vi "UHR-Fleezers Control (host) - 12.8.1.vi"() -> ()   [LabVIEW 2012] (continued)
      }
    }
    n3050 = Negate(x=w3835) -> (-x=w3648:dbl[])
    n3051 = Subtract(x=w3648, y="Offset (nm)") -> (x-y=w3809:dbl[])
    n3052 = case "Choose calibrated display" shown="2" "Calibration" {
      tunnel: w3579 -> [w4240 _ _]
      tunnel: w3576 -> [w4239 _ _]
      tunnel: [w4240 w4242 w4244] -> w3848
      tunnel: [w4239 w4241 w4243] -> w3847
      tunnel: w3578 -> [_ w4242 _]
      tunnel: w3577 -> [_ _ w4244]
      tunnel: w3575 -> [_ w4241 _]
      tunnel: w3574 -> [_ _ w4243]
      frame 0, Default {
      }
      frame 1 {
      }
      frame 2 {
      }
    }
    n3053 = Bundle By Name(cluster=w3579, "Y"=w3809) -> (w3573:waveform(dbl))
    "Bead Separation" <- w3573
    n3054 = feedback #24(w3809) -> (w3808:dbl[])
    n3055 = Build Array (concatenate)(w3809, w3808) -> (w3585:dbl[])
    n3056 = Split 1D Array(array=w3585, index=w3708) -> (first subarray=w3586:dbl[])  [unwired: 1 out]
    n3057 = feedback-in #24(w3586) -> ()
    n3058 = Build Array(w3579, w3578, w3577, w3576, w3575, w3574, w3573) -> (w3572:waveform(dbl)[])
    n3059 = Not(x="Trap Trig. Fl.") -> (.not. x?=w3684:bool)
    n3060 = Unbundle By Name(w3848) -> ("Y"=w3649:dbl[])
    n3061 = Unbundle By Name(w3847) -> ("Y"=w3810:dbl[])
    n3062 = call-poly <vilib>:"Mean.vi"("X"=w3586) -> ("mean"=w3805:dbl)  [unwired: 1 out]
    "Bead Mean (nm)" <- w3805
    n3063 = Multiply(x=w3847, y=-1.0) -> (x*y=w3837:waveform(dbl))
    n3064 = call-poly <vilib>:"Mean.vi"("X"=w3649) -> ("mean"=w3652:dbl)  [unwired: 1 out]
    "T1 X" <- w3652
    n3065 = call-poly <vilib>:"Mean.vi"("X"=w3810) -> ("mean"=w3651:dbl)  [unwired: 1 out]
    "T2 X" <- w3651
    n3066 = Build Array(w3848, w3837) -> (→"Force":waveform(dbl)[])
    n3067 = Subtract(x=w3586, y=w3805) -> (x-y=w3804:dbl[])
    n3068 = Square(x=w3804) -> (x^2=w3803:dbl[])
    n3069 = Negate(x=w3810) -> (-x=w3598:dbl[])
    n3070 = call-poly <vilib>:"Mean.vi"("X"=w3803) -> ("mean"=w3802:dbl)  [unwired: 1 out]
    n3071 = Negate(x=w3651) -> (-x=w3650:dbl)
    n3072 = Square Root(x=w3802) -> (sqrt(x)=w3801:dbl)
    n3073 = Add(x=w3649, y=w3598) -> (x+y=w3811:dbl[])
    n3074 = Add(x=w3652, y=w3650) -> (x+y=w3842:dbl)
    n3075 = Multiply(x=10.0, y=w3801) -> (x*y=→"RMS (Ang)":dbl)
    n3076 = Divide(x=w3811, y=2.0) -> (x/y=w3601:dbl[])
    n3077 = Subtract(x=w3652, y=w3650) -> (x-y=→"Difference":dbl)
    n3078 = Select(t=w3598, s="Only check fixed trap T2", f=w3601) -> (s? t:f=→"Vec Mean of T1 T2":dbl[])
    n3079 = Divide(x=w3842, y=2.0) -> (x/y=w3813:dbl)
    "Mean" <- w3813
    n3080 = feedback-in #25("Trap Trig. Fl.") -> ()
    n3081 = feedback #25("Trap Trig. Fl.") -> (w3682:bool)
    n3082 = And(x=w3684, y=w3682) -> (x .and. y?=w3683:bool)
    n3083 = case "If have just turned off triggering" shown="True" w3683 {
      tunnel: w3665 -> [_ w4040]
      tunnel: w3664 -> [_ w4039]
      frame False {
      }
      frame True {
        w4038 = FALSE ("FPGA Trap Trig")
        n3084 = xnode "Read/Write Control"("FPGA VI Reference In"=w4040, "error in"=w4039, "FPGA Trap Trig"=w4038) -> ("FPGA VI Reference Out"=w4037:T24, "error out"=w4036:errorcluster)
        n3085 = xnode "Read/Write Control"("FPGA VI Reference In"=w4037, "error in"=w4036, "TTrig?"=w4038) -> ()  [unwired: 2 out]
        n3086 = local write "Initializing"(FALSE ("Initializing")) -> ()
        n3087 = local write "Triggered"(FALSE ("Triggered")) -> ()
        n3088 = local write "Waiting"(FALSE ("Waiting")) -> ()
      }
    }
    n3089 = Not(x=w3682) -> (.not. x?=w3695:bool)
    n3090 = And(x="Trap Trig. Fl.", y=w3695) -> (x .and. y?=w3692:bool)
    n3091 = Or(x=w3692, y="Reinitialize") -> (x .or. y?=w3678:bool)
    n3092 = feedback #26(w3688) -> (w3693:string)
    n3093 = Select(t=w3688, s=w3692, f=w3693) -> (s? t:f=w3687:string)
    n3094 = Select(t=w3688, s="Reinitialize", f=w3687) -> (s? t:f=w3686:string)
    n3095 = local read "Tether"() -> (w3814:bool)
    n3096 = feedback #27(0) -> (w3690:i32)
    n3097 = case "For determining if there is a tether still" shown="True" w3814 {
      tunnel: w3813 -> [_ w4164]
      frame False {
      }
      frame True {
        n3098 = Greater?(x="Lost Tether Alarm Threshold (pN)", y=w4164) -> (0:w4162:bool)
        n3099 = case shown="True" w4162 {
          frame False {
          }
          frame True {
            w4165 = FALSE ("Value (Signaling)")
            n3100 = flat-sequence {
              frame #0 {
                # "stop only if saving"
                n3101 = local read "Saving..."() -> (w4177:bool)
                n3102 = And(x=w4177, y="TA Cancel Save?") -> (x .and. y?=w4176:bool)
                n3103 = local write "Stop Saving"(w4176) -> ()
              }
              frame #1 {
                n3104 = case shown="True" "TA Green Off?" {
                  frame False {
                  }
                  frame True {
                    w4180 = FALSE ("Fl. Triggered...")
                    n3105 = local write "Fl. Triggered..."(w4180) -> ()
                    n3106 = property on="Green Laser ON" class="Bool (strict)"("Val(Sgnl)"=w4180) -> ()  [unwired: 2 in, 2 out]
                  }
                }
              }
            }
            n3107 = local read "Time tether formed"() -> (w4171:timestamp)
            n3108 = Get Date/Time In Seconds() -> (seconds since 1Jan1904=w4172:timestamp)
            n3109 = Subtract(x=w4172, y=w4171) -> (x-y=w4170:dbl)
            n3110 = Number To Decimal String(number=w4170) -> (decimal integer string=w4167:string)  [unwired: 1 out]
            n3111 = local read "Messages"() -> (w4174:string)
            n3112 = call <vilib>:"Beep.vi"() -> ()  [unwired: 3 in, 9 out]
            n3113 = Concatenate Strings("Lost tether (" ("Message to add"), w4167, " s)." ("string")) -> (w4169:string)
            n3114 = local write "Tether"(FALSE ("Tether")) -> ()
            n3115 = call "Update messages.vi"("Message to add"=w4169, "Old message string"=w4174) -> ("New message string"=w4173:string)
            n3116 = local write "Messages"(w4173) -> ()
            n3117 = property on="Fl. Triggered..." class="Bool (strict)"("Val(Sgnl)"=w4165) -> ()  [unwired: 2 in, 2 out]
            n3118 = local write "Dip for Protein"(w4165) -> ()
            n3119 = property on="Trap Pos. FB ON" class="Bool (strict)"("Val(Sgnl)"=w4165) -> ()  [unwired: 2 in, 2 out]
            n3120 = property on="Trap Trig. Fl." class="Bool (strict)"("Val(Sgnl)"=w4165) -> ()  [unwired: 2 in, 2 out]
          }
        }
      }
    }
    n3121 = case "For triggering actions based on the trap position (e.g., turning the excitation laser on if trap under feedback moves so far)" shown="True" "Trap Trig. Fl." {
      tunnel: w3673 -> [_ w4053]
      tunnel: w3686 -> [_ w4052]
      tunnel: ["" ("t") w4051] -> w3694
      tunnel: w3678 -> [_ w4050]
      tunnel: [0 ("t") w4049] -> w3691
      tunnel: w3690 -> [_ w4048]
      tunnel: w3665 -> [_ w4047]
      tunnel: w3664 -> [_ w4046]
      frame False {
      }
      frame True {
        n3122 = case shown="\"Wait for trigger\"" w4052 {
          tunnel: w4053 -> [w4070 _ _ w4118]
          tunnel: [w4067 w4099 "" ("t") w4121] -> w4051
          tunnel: w4050 -> [_ _ _ w4109]
          tunnel: [w4066 w4096 0 ("t") w4110] -> w4049
          tunnel: w4048 -> [_ w4098 _ w4116]
          tunnel: w4047 -> [w4055 w4093 _ w4112]
          tunnel: w4046 -> [w4054 w4092 _ w4111]
          frame "Wait for trigger" {
            n3123 = local read "Trap Trig. (FPGA)"() -> (w4058:bool)
            n3124 = Subtract(x=w4070, y="Mean T1 Position\nto compare (nm)") -> (x-y=w4063:dbl[])
            n3125 = call <vilib>:"Std Deviation and Variance.vi"("X"=w4063) -> ("mean"=→"mean":dbl, "standard deviation"=→"standard\ndeviation":dbl)  [unwired: 1 in, 1 out]
            n3126 = Array Max & Min(array=w4063) -> (max value=→"max value":dbl, min value=→"min value":dbl)  [unwired: 2 out]
            n3127 = Greater?(x=w4063, y="Threshold (nm)") -> (0:w4073:bool[])
            n3128 = case shown="True" w4058 {
              tunnel: w4055 -> [_ w4079]
              tunnel: w4054 -> [_ w4078]
              tunnel: [FALSE ("TTrig?") w4077] -> w4061
              frame False {
              }
              frame True {
                n3129 = xnode "Read/Write Control"("FPGA VI Reference In"=w4079, "error in"=w4078) -> ("TTrig?"=w4077:bool)  [unwired: 2 out]
              }
            }
            n3130 = Or Array Elements(Boolean array=w4073) -> (logical OR=w4060:bool)
            n3131 = Select(t=w4061, s=w4058, f=w4060) -> (s? t:f=w4059:bool)
            n3132 = Not(x=w4058) -> (.not. x?=w4057:bool)
            n3133 = And(x=w4059, y=w4057) -> (x .and. y?=w4056:bool)
            n3134 = Select(t="Triggered", s=w4059, f="Wait for trigger") -> (s? t:f=w4067:string)
            n3135 = case shown="True" w4059 {
              tunnel: [0 0] -> w4066
              tunnel: w4055 -> [_ w4084]
              tunnel: w4054 -> [_ w4083]
              frame False {
                "Waiting" <- TRUE ("Waiting")
              }
              frame True {
                n3136 = xnode "Read/Write Control"("FPGA VI Reference In"=w4084, "error in"=w4083, "TTrig?"=FALSE) -> ()  [unwired: 2 out]
                n3137 = local read "Messages"() -> (w4087:string)
                n3138 = call <vilib>:"Beep.vi"() -> ()  [unwired: 12 in]
                n3139 = call "Update messages.vi"("Message to add"="Unwinding trigger.", "Old message string"=w4087) -> ("New message string"=w4088:string)
                n3140 = local write "Messages"(w4088) -> ()
                n3141 = local write "Waiting"(FALSE ("Waiting")) -> ()
                "Triggered" <- TRUE ("Triggered")
              }
            }
            n3142 = case "Only need to turn on laser if host triggered" shown="True" w4056 {
              frame False {
              }
              frame True {
                n3143 = property on="Green Laser ON" class="Bool (strict)"("Val(Sgnl)"=TRUE ("Value (Signaling)")) -> ()  [unwired: 2 in, 2 out]
              }
            }
          }
          frame "Triggered" {
            n3144 = local read "Trap Trig. (FPGA)"() -> (w4095:bool)
            n3145 = Increment(x=w4098) -> (x+1=w4096:i32)
            n3146 = Greater Or Equal?(x=w4096, y="Fl. ON time (n)") -> (x >= y?=w4094:bool)
            n3147 = Select(t="Wait for trigger", s=w4094, f="Triggered" ("t")) -> (s? t:f=w4099:string)
            n3148 = And(x=w4094, y=w4095) -> (x .and. y?=w4091:bool)
            n3149 = case shown="True" w4091 {
              tunnel: w4093 -> [_ w4103]
              tunnel: w4092 -> [_ w4102]
              frame False {
              }
              frame True {
                n3150 = xnode "Read/Write Control"("FPGA VI Reference In"=w4103, "error in"=w4102, "FPGA Trap Trig"=TRUE) -> ()  [unwired: 2 out]
              }
            }
            n3151 = case shown="True" w4094 {
              frame False {
              }
              frame True {
                w4105 = FALSE ("Value (Signaling)")
                n3152 = local write "Triggered"(w4105) -> ()
                n3153 = local write "Waiting"(TRUE ("Waiting")) -> ()
                n3154 = property on="Green Laser ON" class="Bool (strict)"("Val(Sgnl)"=w4105) -> ()  [unwired: 2 in, 2 out]
              }
            }
          }
          frame "Do nothing" {
          }
          frame "Initialize", Default {
            n3155 = Increment(x=w4116) -> (x+1=w4120:i32)
            n3156 = Select(t=1, s=w4109, f=w4120) -> (s? t:f=w4110:i32)
            n3157 = feedback #28(w4118) -> (w4124:dbl[])
            n3158 = Build Array (concatenate)(w4118, w4124) -> (w4117:dbl[])
            n3159 = Greater Or Equal?(x=w4110, y="Wait to get offset (n)") -> (x >= y?=w4113:bool)
            n3160 = Select(t=w4118, s=w4109, f=w4117) -> (s? t:f=w4119:dbl[])
            n3161 = feedback-in #28(w4119) -> ()
            n3162 = call-poly <vilib>:"Mean.vi"("X"=w4119) -> ("mean"=w4114:dbl)  [unwired: 1 out]
            n3163 = local write "Mean T1 Position\nto compare (nm)"(w4114) -> ()
            n3164 = case shown="True" w4109 {
              tunnel: w4112 -> [_ w4130]
              tunnel: w4111 -> [_ w4129]
              frame False {
              }
              frame True {
                w4126 = FALSE ("FPGA Trap Trig")
                n3165 = xnode "Read/Write Control"("FPGA VI Reference In"=w4130, "error in"=w4129, "FPGA Trap Trig"=w4126) -> ("FPGA VI Reference Out"=w4128:T24, "error out"=w4127:errorcluster)
                n3166 = xnode "Read/Write Control"("FPGA VI Reference In"=w4128, "error in"=w4127, "TTrig?"=w4126) -> ()  [unwired: 2 out]
              }
            }
            n3167 = Select(t="Wait for trigger", s=w4113, f="Initialize") -> (s? t:f=w4121:string)
            n3168 = case shown="True" w4113 {
              tunnel: w4114 -> [_ w4133]
              tunnel: w4112 -> [_ w4142]
              tunnel: w4111 -> [_ w4141]
              frame False {
                n3169 = local write "Waiting"(FALSE ("Waiting")) -> ()
                "Initializing" <- TRUE ("Initializing")
              }
              frame True {
                n3170 = local read "Threshold (nm)"() -> (w4145:dbl)
                n3171 = local read "AOM X Cal (nm/MHz)"() -> (w4144:dbl)
                n3172 = Add(x=w4133, y=w4145) -> (x+y=w4146:dbl)
                n3173 = Divide(x=w4146, y=w4144) -> (x/y=w4143:dbl)
                n3174 = call "IR AOM freq to word.vi"("Frequency In (MHz)"=w4143) -> ("Frequency Word Out (double)"=w4140:dbl)
                n3175 = local write "Initializing"(FALSE ("Initializing")) -> ()
                n3176 = local write "Waiting"(TRUE ("Waiting")) -> ()
                n3177 = To Quad Integer(1:w4140) -> (0:w4139:i64)
                n3178 = xnode "Read/Write Control"("FPGA VI Reference In"=w4142, "error in"=w4141, "FPGA TTrig Thresh"=w4139) -> ("FPGA VI Reference Out"=w4136:T24, "error out"=w4135:errorcluster)
                n3179 = xnode "Read/Write Control"("FPGA VI Reference In"=w4136, "error in"=w4135, "FPGA Trap Trig"=TRUE) -> ()  [unwired: 2 out]
              }
            }
          }
        }
      }
    }
    n3180 = feedback-in #26(w3694) -> ()
    n3181 = feedback-in #27(w3691) -> ()
    n3182 = xnode ("Read/Write Control")("FPGA VI Reference In"=w3833, "error in"=w3832) -> ("FPGA VI Reference Out"=w3676:T24, "error out"=w3675:errorcluster, "AI2 Y Sum Set 1"=w3907:i16, "AI2 Y Sum Set 2"=w3906:i16, "AI1 X Set 1"=w3740:fxp<+/-,16,1>, "AI1 X Set 2"=w3739:fxp<+/-,16,1>, "Trap Pos FB Int Signal"=→"Trap Pos FB Int Signal":fxp<+/-,24,9>, "Trap Pos FB Int-Norm Signal"=→"Trap Pos FB Int-Norm Signal":fxp<+/-,16,1>, "Trap Pos FB Action"=w3733:i64, "Scanning"=→"AOD Scanning":bool, "Scan I"=→"AOD Scan I":u64, "Scanning MCL"=w3909:bool, "Scan I (MCL)"=→"MCL Scan I":u64, "Green FB Sum"=w3849:i16, "Trap Pos FB Action"=w3663:i64, "TTrig Fin Thresh"=w3659:i64, "Red FB Intensity"=w3643:i16, "Blue Intensity"=w3638:i16)
    "MCL Scanning" <- w3909
    "Trap Pos FB Action" <- w3733
    n3183 = Divide(x=w3643, y=3276.7) -> (x/y=w3642:dbl)
    "Red laser intensity (V)" <- w3642
    n3184 = Divide(x=w3638, y=3276.7) -> (x/y=w3637:dbl)
    "Blue laser intensity (V)" <- w3637
    n3185 = Divide(x=w3849, y=3276.7) -> (x/y=w3641:dbl)
    "Green laser intensity (V)" <- w3641
    n3186 = local read "FB Trig Integrate"() -> (w3657:u32)
    n3187 = Divide(x=w3663, y=w3657) -> (x/y=w3656:dbl)
    "TTrig Sig (Int)" <- w3656
    n3188 = Bundle(w3641, w3642, w3637) -> (→"Fluorescence laser intensities plot":cluster{dbl, dbl, dbl})  [unwired: 1 in]
    n3189 = Divide(x=w3659, y=w3657) -> (x/y=w3654:dbl)
    "TTrig Fin Thresh (Int)" <- w3654
    n3190 = local read "AOM X Cal (nm/MHz)"() -> (w3662:dbl)
    n3191 = local read "AI2 (V)"() -> (w3908:cluster{"Set 1":dbl, "Set 2":dbl})
    n3192 = Bundle By Name(cluster=w3908, "Set 1"=w3907, "Set 2"=w3906) -> (w3904:cluster{"Set 1":dbl, "Set 2":dbl})
    n3193 = Divide(x=w3733, y=327.67) -> (x/y=→"Action (%)":dbl)
    n3194 = local read "Trap X (AI1)"() -> (w3753:T12)
    n3195 = call "IR AOM word double to freq.vi"("Frequency Word In (double)"=w3654) -> ("Frequency Out (MHz)"=w3653:dbl)
    n3196 = call "IR AOM word double to freq.vi"("Frequency Word In (double)"=w3656) -> ("Frequency Out (MHz)"=w3655:dbl)
    n3197 = Divide(x=w3904, y=3276.7) -> (x/y=w3903:cluster{"Set 1":dbl, "Set 2":dbl})
    n3198 = Multiply(x=w3655, y=w3662) -> (x*y=w3661:dbl)
    "TTrig Sig (nm)" <- w3661
    n3199 = Multiply(x=w3653, y=w3662) -> (x*y=w3660:dbl)
    "TTrig Fin Thresh (nm)" <- w3660
    n3200 = local write "AI2 (V)"(w3903) -> ()
    n3201 = Bundle(cluster=w3753, "Trap 1"=w3740, "Trap 2"=w3739) -> (→"Trap X (AI1)":T12)
    n3202 = Bundle(w3661, w3660) -> (→"TTrig":cluster{dbl, dbl})  [unwired: 1 in]
    n3203 = flat-sequence "To save data" {
      tunnel: [w5009] -> w3927
      tunnel: [w5010] -> w3926
      tunnel: w3878 -> [w5003]
      tunnel: w3681 -> [w5007]
      tunnel: ["Save Calibration"] -> w3900
      tunnel: w3897 -> [w5006]
      tunnel: [w4999] -> w3896
      tunnel: [w4996] -> w3895
      tunnel: [w4993] -> w3894
      tunnel: w3877 -> [w4995]
      tunnel: w3817 -> [w4989]
      tunnel: [w4989] -> w3816
      tunnel: [w4981] -> w3790
      tunnel: [w4984] -> w3721
      tunnel: [w4983] -> w3720
      tunnel: w3927 -> [w5259]
      tunnel: w3926 -> [w5258]
      tunnel: w3722 -> [w5257]
      tunnel: w3900 -> [w5256]
      tunnel: w3896 -> [w5254]
      tunnel: w3895 -> [w5253]
      tunnel: w3894 -> [w5252]
      tunnel: w3798 -> [w5251]
      tunnel: w3825 -> [w5250]
      tunnel: w3816 -> [w5249]
      tunnel: w3790 -> [w5248]
      tunnel: w3573 -> [w5247]
      tunnel: w3623 -> [w5246]
      tunnel: w3721 -> [w5245]
      tunnel: w3720 -> [w5244]
      tunnel: w3719 -> [w5243]
      tunnel: w3645 -> [w5242]
      frame #0 {
        n3204 = Or(x="Start Saving", y="Start saving data + video") -> (x .or. y?=w4981:bool)
        n3205 = case shown="True" "Start saving data + video" {
          frame False {
          }
          frame True {
            n3206 = stacked-sequence {
              frame #0 {
                n3207 = local write "New Video File"(TRUE ("New Video File")) -> ()
              }
              frame #1 {
                n3208 = local write "Save Video"(TRUE ("Save Video")) -> ()
              }
            }
          }
        }
        n3209 = Or(x="Save N Sets", y=w4981) -> (x .or. y?=w4990:bool)
        n3210 = To Double Precision Float(number=w5006) -> (double precision float=w5000:dbl)
        n3211 = Build Array(w4990, "Save Calibration", w5003, w4995) -> (w5005:bool[])
        n3212 = Compound Arithmetic op=OR("Save Calibration", w5003, w4990, w4995) -> (w5008:bool)
        n3213 = Boolean Array To Number(Boolean array=w5005) -> (number=w5002:u32)
        n3214 = feedback #29(FALSE ("Save APD Data\nwith Trap Data")) -> (w4985:bool)
        n3215 = feedback #30(refnum<k0> refnum) -> (w5011:refnum<file>)
        n3216 = feedback #31(refnum<k0> refnum) -> (w4987:refnum<file>)
        n3217 = feedback #32(FALSE ("Save APD Data\nwith Trap Data")) -> (w4994:bool)
        n3218 = feedback #33(refnum<k0> refnum) -> (w4997:refnum<file>)
        n3219 = feedback #34(0) -> (w5013:i32)
        n3220 = feedback #35() -> (w5001:u32)  [unwired: 1 out]
        n3221 = case shown="True" w5008 {
          tunnel: [w5022 1] -> w5009
          tunnel: w5013 -> [w5024 _]
          tunnel: [w5023 w5055] -> w5010
          tunnel: w5011 -> [w5023 _]
          tunnel: w5007 -> [_ w5073]
          tunnel: w5000 -> [_ w5071]
          tunnel: w5002 -> [_ w5074]
          tunnel: [w5021 w5054] -> w4999
          tunnel: w5001 -> [w5021 _]
          tunnel: [w5020 w5052] -> w4996
          tunnel: w4997 -> [w5020 _]
          tunnel: [w5019 w5051] -> w4993
          tunnel: w4994 -> [w5019 _]
          tunnel: w4981 -> [_ w5049]
          tunnel: w4989 -> [_ w5048]
          tunnel: [w5018 w5040] -> w4983
          tunnel: w4987 -> [w5018 _]
          tunnel: [w5017 w5039] -> w4984
          tunnel: w4985 -> [w5017 _]
          frame False {
            n3222 = Increment(x=w5024) -> (x+1=w5022:i32)
          }
          frame True {
            w5045 = FALSE ("Start Saving")
            w5050 = 9.0  # File Version
            w5057 = FALSE ("prepend array or string size? (T)")
            w5056 = T32."big-endian, network order" ("byte order (0:big-endian, network order)")
            n3223 = local read "BD 1 Frequency 1 (MHz)"() -> (w5070:dbl)
            n3224 = local read "BD 2 Frequency 1 (MHz)"() -> (w5069:dbl)
            n3225 = local read "BD 1 Frequency 2 (MHz)"() -> (w5068:dbl)
            n3226 = local read "BD 2 Frequency 2 (MHz)"() -> (w5067:dbl)
            n3227 = local read "BD 1 Frequency 3 (MHz)"() -> (w5066:dbl)
            n3228 = local read "BD 2 Frequency 3 (MHz)"() -> (w5065:dbl)
            n3229 = Array Size(array=w5048) -> (size(s)=w5047:i32)
            n3230 = To Double Precision Float(number=w5047) -> (double precision float=w5046:dbl)
            n3231 = local write "Save Calibration"(w5045) -> ()
            n3232 = local write "Start Saving"(w5045) -> ()
            n3233 = Build Array("Save APD Data\nwith Trap Data", "Save Trap Pos. Data") -> (w5042:bool[])
            n3234 = Boolean Array To Number(Boolean array=w5042) -> (number=w5041:u32)
            n3235 = Build Array(w5070, w5069, w5068, w5067, w5066, w5065) -> (w5064:dbl[])
            n3236 = case shown="1, Default" w5074 {
              tunnel: w5073 -> [w5146 w5166 w5182 w5220]
              tunnel: w5046 -> [w5151 w5173 w5202 w5239]
              tunnel: w5071 -> [w5150 w5172 w5201 w5238]
              tunnel: [w5147 w5168 w5193 w5230] -> w5062
              tunnel: [w5138 "Cal sets to save" w5183 w5221] -> w5054
              tunnel: w5064 -> [w5148 w5169 w5195 w5232]
              tunnel: "Save APD Data\nwith Trap Data" -> [w5145 _ w5179 w5218]
              tunnel: [w5145 w5160 w5179 w5218] -> w5051
              tunnel: w5050 -> [w5141 w5161 w5177 w5216]
              tunnel: w5049 -> [w5140 _ _ _]
              tunnel: [w5131 w5160 w5176 w5206] -> w5039
              tunnel: "Save Trap Pos. Data" -> [w5131 _ w5176 w5206]
              tunnel: w5041 -> [w5130 _ w5175 w5205]
              frame 1, Default {
                # "timeseries"
                n3237 = case shown="True" "Profile" {
                  tunnel: [w5154 w5158] -> w5135
                  tunnel: [w5154 w5157] -> w5134
                  tunnel: [w5154 w5156] -> w5133
                  tunnel: [w5154 w5155] -> w5132
                  frame False {
                    w5154 = 0.0 ("f")
                  }
                  frame True {
                    n3238 = local read "Current Position"() -> (w5159:cluster{dbl, dbl, dbl})
                    n3239 = local read "Y change (mm)"() -> (w5155:dbl)
                    n3240 = Unbundle(w5159) -> (w5158:dbl, w5157:dbl, w5156:dbl)
                  }
                }
                n3241 = local read "Save ave N"() -> (w5153:dbl)
                n3242 = Multiply(x=w5153, y=w5146) -> (x*y=w5152:dbl)
                n3243 = To Double Precision Float(number=w5130) -> (double precision float=w5144:dbl)
                n3244 = Build Array(w5141, w5146, w5152, w5151, w5150, 0.0 ("f")) -> (w5149:dbl[])
                n3245 = Build Array(w5144, w5135, w5134, w5133, w5132) -> (w5142:dbl[])
                n3246 = Select(t=u32 4000000000, s=w5140, f="N sets to save") -> (s? t:f=w5138:u32)
                n3247 = Build Array (concatenate)(w5149, w5148, w5142) -> (w5147:dbl[])
              }
              frame 2 {
                w5163 = 0.0 ("f")
                w5160 = FALSE ("Save APD Data\nwith Trap Data")
                # "calibration"
                n3248 = Boolean To (0,1)(Boolean=w5160) -> (0, 1=w5165:i16)
                n3249 = To Double Precision Float(number=w5165) -> (double precision float=w5164:dbl)
                n3250 = Build Array(w5164, w5163, w5163, w5163, w5163) -> (w5162:dbl[])
                n3251 = Build Array(w5161, w5166, w5166, w5173, w5172, 1.0 ("t")) -> (w5170:dbl[])
                n3252 = Build Array (concatenate)(w5170, w5169, w5162) -> (w5168:dbl[])
                "Calibrating Trap..." <- TRUE ("Calibrating...")
              }
              frame 4 {
                w5180 = 0.0 ("f")
                # "scan dir (x/y = 0/1)"
                # "cycles/step"
                # "n scans (f/b)"
                # "steps"
                # "freq. range"
                # "AOD raster scan"
                n3253 = local read "Number of F/B Scans (AOD)"() -> (w5187:u16)
                n3254 = local read "Cycles/step (AOD)"() -> (w5189:u64)
                n3255 = local read "Scan Range (MHz)"() -> (w5192:dbl)
                n3256 = local read "Scan steps (AOD)"() -> (w5191:u64)
                n3257 = local read "Scan BD"() -> (w5199:bool)
                n3258 = local read "Save ave N"() -> (w5204:dbl)
                n3259 = Boolean To (0,1)(Boolean=w5199) -> (0, 1=w5198:i16)
                n3260 = To Double Precision Float(number=w5187) -> (double precision float=w5186:dbl)
                n3261 = To Double Precision Float(number=w5191) -> (double precision float=w5190:dbl)
                n3262 = To Double Precision Float(number=w5189) -> (double precision float=w5188:dbl)
                n3263 = To Double Precision Float(number=w5198) -> (double precision float=w5197:dbl)
                n3264 = Multiply(x=w5204, y=w5182) -> (x*y=w5203:dbl)
                n3265 = To Double Precision Float(number=w5175) -> (double precision float=w5181:dbl)
                n3266 = Build Array(w5181, w5180, w5180, w5180, w5180) -> (w5178:dbl[])
                n3267 = local read "N sets should be saved"() -> (w5184:dbl)
                n3268 = Build Array(w5197, w5192, w5190, w5188, w5186) -> (w5194:dbl[])
                n3269 = Build Array(w5177, w5182, w5203, w5202, w5201, 2.0 ("t")) -> (w5196:dbl[])
                n3270 = Round Toward +Infinity(x=w5184) -> (ceil(x): smallest int >= x=w5185:dbl)
                n3271 = Build Array (concatenate)(w5196, w5195, w5178, w5194) -> (w5193:dbl[])
                n3272 = To Unsigned Long Integer(number=w5185) -> (unsigned 32bit integer=w5183:u32)
              }
              frame 8 {
                w5213 = 0.0 ("f")
                # "MCL raster scan"
                n3273 = local read "Number of scans (MCL)"() -> (w5208:u64)
                n3274 = local read "Scan lines (y)"() -> (w5207:u64)
                n3275 = local read "2D or 1D Scan"() -> (w5210:bool)
                n3276 = local read "Scan Range (V)\n(of steps)"() -> (w5229:dbl)
                n3277 = local read "Fast Scan Dir"() -> (w5236:bool)
                n3278 = local read "Cycles/step (MCL)"() -> (w5226:u64)
                n3279 = local read "Scan steps (MCL)"() -> (w5228:u64)
                n3280 = Select(t=w5207, s=w5210, f=w5208) -> (s? t:f=w5209:u64)
                n3281 = Boolean To (0,1)(Boolean=w5210) -> (0, 1=w5212:i16)
                n3282 = local read "Save ave N"() -> (w5241:dbl)
                n3283 = local read "Initial X"() -> (w5215:dbl)
                n3284 = local read "Initial Y"() -> (w5214:dbl)
                n3285 = To Double Precision Float(number=w5212) -> (double precision float=w5211:dbl)
                n3286 = Boolean To (0,1)(Boolean=w5236) -> (0, 1=w5235:i16)
                n3287 = To Double Precision Float(number=w5209) -> (double precision float=w5224:dbl)
                n3288 = To Double Precision Float(number=w5228) -> (double precision float=w5227:dbl)
                n3289 = To Double Precision Float(number=w5226) -> (double precision float=w5225:dbl)
                n3290 = To Double Precision Float(number=w5235) -> (double precision float=w5234:dbl)
                n3291 = Multiply(x=w5241, y=w5220) -> (x*y=w5240:dbl)
                n3292 = To Double Precision Float(number=w5205) -> (double precision float=w5219:dbl)
                n3293 = local read "N sets should be saved (MCL)"() -> (w5222:dbl)
                n3294 = Build Array(w5219, w5211, w5213, w5213, w5213) -> (w5217:dbl[])
                n3295 = Build Array(w5234, w5229, w5227, w5225, w5224, w5215, w5214) -> (w5231:dbl[])
                n3296 = Build Array(w5216, w5220, w5240, w5239, w5238, 3.0 ("t")) -> (w5233:dbl[])
                n3297 = Round Toward +Infinity(x=w5222) -> (ceil(x): smallest int >= x=w5223:dbl)
                n3298 = Build Array (concatenate)(w5233, w5232, w5217, w5231) -> (w5230:dbl[])
                n3299 = To Unsigned Long Integer(number=w5223) -> (unsigned 32bit integer=w5221:u32)
              }
            }
            n3300 = local read "Index"() -> (w5079:dbl)
            n3301 = call "Create new save file.vi"("Insert"="", "Ext"=".dat", "Index In"=w5079) -> ("Path Out"=w5035:path, "Index Out"=w5053:dbl)
            n3302 = local write "Save file name"(w5035) -> ()
            n3303 = local write "Index"(w5053) -> ()
            n3304 = local write "Save index"(w5053) -> ()
            n3305 = Array Size(array=w5062) -> (size(s)=w5063:i32)
            n3306 = Open/Create/Replace File(file path (use dialog)=w5035, operation (0:open)=T33."create", access (0:read/write)=enum16{"read/write", "read-only", "write-only"}."write-only") -> (refnum out=w5076:refnum<file>)  [unwired: 1 in, 4 out]
            n3307 = local write "Saving..."(TRUE ("Saving...")) -> ()
            n3308 = To Double Precision Float(number=w5063) -> (double precision float=w5061:dbl)
            n3309 = String Length(string="Comment (data description)") -> (length=w5060:i32)
            n3310 = To Double Precision Float(number=w5060) -> (double precision float=w5059:dbl)
            n3311 = Deny Access(7:w5076) -> (3:w5075:refnum<file>)  [unwired: 1 in, 2 out]
            n3312 = Build Array (concatenate)(w5061, w5062, w5059) -> (w5034:dbl[])
            n3313 = case "If fluorescence data to be saved" shown="True" w5051 {
              tunnel: w5035 -> [_ w5129]
              tunnel: [refnum<k0> refnum w5109] -> w5052
              frame False {
              }
              frame True {
                w5108 = 0.0
                n3314 = local read "APD Integration Time (s)"() -> (w5114:dbl)
                n3315 = local read "N APD Samp/step"() -> (w5107:dbl)
                n3316 = local read "Number of APDs"() -> (w5106:u8)
                n3317 = Path To String(path=w5129) -> (string=w5128:string)
                n3318 = String Length(string=w5128) -> (length=w5127:i32)
                n3319 = Subtract(x=w5127, y=4) -> (x-y=w5125:i32)
                n3320 = String Subset(string=w5128, length (rest)=w5125) -> (substring=w5124:string)  [unwired: 1 out]
                n3321 = Build Array(w5114, w5107, w5106, w5108, w5108, w5108, w5108, w5108) -> (w5111:dbl[])
                n3322 = Concatenate Strings(w5124, "_fl.dat" ("string")) -> (w5122:string)
                n3323 = Array Size(array=w5111) -> (size(s)=w5113:i32)
                n3324 = String To Path(string=w5122) -> (path=w5118:path)
                n3325 = Open/Create/Replace File(file path (use dialog)=w5118, operation (0:open)=T33."create", access (0:read/write)=enum16{"read/write", "read-only", "write-only"}."write-only") -> (refnum out=w5119:refnum<file>)  [unwired: 1 in, 4 out]
                n3326 = Deny Access(7:w5119) -> (3:w5115:refnum<file>)  [unwired: 1 in, 2 out]
                n3327 = To Double Precision Float(number=w5113) -> (double precision float=w5112:dbl)
                n3328 = Build Array (concatenate)(w5112, w5111) -> (w5110:dbl[])
                n3329 = Write to Binary File(file (use dialog)=w5115, data=w5110, 5:FALSE ("prepend array or string size? (T)"), 9:T32."big-endian, network order" ("byte order (0:big-endian, network order)")) -> (refnum out=w5109:refnum<file>)  [unwired: 1 in, 3 out]
              }
            }
            n3330 = case shown="True" w5039 {
              tunnel: w5035 -> [_ w5090]
              tunnel: [refnum<k0> refnum w5089] -> w5040
              frame False {
              }
              frame True {
                w5085 = 0.0 ("element")
                n3331 = Path To String(path=w5090) -> (string=w5104:string)
                n3332 = Build Array(w5085, w5085, w5085, w5085, w5085, w5085, w5085, w5085) -> (w5086:dbl[])
                n3333 = String Length(string=w5104) -> (length=w5103:i32)
                n3334 = Subtract(x=w5103, y=4) -> (x-y=w5101:i32)
                n3335 = Array Size(array=w5086) -> (size(s)=w5088:i32)
                n3336 = String Subset(string=w5104, length (rest)=w5101) -> (substring=w5100:string)  [unwired: 1 out]
                n3337 = To Double Precision Float(number=w5088) -> (double precision float=w5087:dbl)
                n3338 = Concatenate Strings(w5100, "_pos.dat" ("string")) -> (w5098:string)
                n3339 = Build Array (concatenate)(w5087, w5086) -> (w5084:dbl[])
                n3340 = String To Path(string=w5098) -> (path=w5094:path)
                n3341 = Open/Create/Replace File(file path (use dialog)=w5094, operation (0:open)=T33."create", access (0:read/write)=enum16{"read/write", "read-only", "write-only"}."write-only") -> (refnum out=w5095:refnum<file>)  [unwired: 1 in, 4 out]
                n3342 = Deny Access(7:w5095) -> (3:w5091:refnum<file>)  [unwired: 1 in, 2 out]
                n3343 = Write to Binary File(file (use dialog)=w5091, data=w5084, 5:FALSE ("prepend array or string size? (T)"), 9:T32."big-endian, network order" ("byte order (0:big-endian, network order)")) -> (refnum out=w5089:refnum<file>)  [unwired: 1 in, 3 out]
              }
            }
            n3344 = Write to Binary File(file (use dialog)=w5075, data=w5034, 5:w5057, 9:w5056) -> (refnum out=w5058:refnum<file>)  [unwired: 1 in, 3 out]
            n3345 = Write to Binary File(file (use dialog)=w5058, data="Comment (data description)", 5:w5057, 9:w5056) -> (refnum out=w5055:refnum<file>)  [unwired: 1 in, 3 out]
            n3346 = local read "connection reference"() -> (w5037:T19)
            n3347 = Bundle("Comment (data description)"="Comment (data description)", "Channel 1 Buffer"="Channel 1 Buffer", "Channel 2 Buffer"="Channel 2 Buffer", "Channel 3 Buffer"="Channel 3 Buffer", "Title"="Title", "DNA Construct"="DNA Construct", "Bead diameter"="Bead diameter", "Name"="Name") -> (w5025:T55)  [unwired: 1 in]
            n3348 = call "MattFileCreator-v9.vi"("Comments"=w5025, "Input Array"=w5034, "File path"=w5035, "table"="labview", "connection reference"=w5037) -> ("connection reference out"=w5036:T19)  [unwired: 5 in, 1 out]
            n3349 = local write "connection reference"(w5036) -> ()
          }
        }
        n3350 = feedback-in #29(w4984) -> ()
        n3351 = feedback-in #30(w5010) -> ()
        n3352 = feedback-in #31(w4983) -> ()
        n3353 = feedback-in #32(w4993) -> ()
        n3354 = feedback-in #33(w4996) -> ()
        n3355 = feedback-in #34(w5009) -> ()
        n3356 = feedback-in #35(w4999) -> ()
      }
      frame #1 {
        n3357 = local read "Saving..."() -> (w5255:bool)
        n3358 = case shown="True" w5255 {
          tunnel: w5259 -> [_ w5271]
          tunnel: w5258 -> [_ w5285]
          tunnel: w5257 -> [_ w5281]
          tunnel: w5256 -> [_ w5280]
          tunnel: w5254 -> [_ w5279]
          tunnel: w5253 -> [_ w5274]
          tunnel: w5252 -> [_ w5273]
          tunnel: w5251 -> [_ w5272]
          tunnel: w5250 -> [_ w5270]
          tunnel: w5249 -> [_ w5268]
          tunnel: w5248 -> [_ w5267]
          tunnel: w5247 -> [_ w5266]
          tunnel: w5246 -> [_ w5265]
          tunnel: w5245 -> [_ w5264]
          tunnel: w5244 -> [_ w5263]
          tunnel: w5243 -> [_ w5262]
          tunnel: w5242 -> [_ w5261]
          frame False {
          }
          frame True {
            n3359 = case shown="True" "Stop saving data + video" {
              frame False {
              }
              frame True {
                n3360 = local write "Save Video"(FALSE ("Save Video")) -> ()
              }
            }
            n3361 = Multiply(x=w5271, y=w5270) -> (x*y=→"Time (s)":dbl)
            n3362 = Less Or Equal?(x=w5271, y=w5279) -> (x <= y?=w5283:bool)
            n3363 = Compound Arithmetic op=OR("Stop Saving", "Abort save 2", "Stop saving data + video") -> (w5275:bool)
            n3364 = Not(x=w5275) -> (.not. x?=w5284:bool)
            n3365 = And(x=w5283, y=w5284) -> (x .and. y?=w5282:bool)
            n3366 = case shown="True" w5282 {
              tunnel: w5285 -> [w5293 w5384]
              tunnel: [0.0 w5387] -> w5278
              tunnel: w5271 -> [_ w5385]
              tunnel: w5279 -> [_ w5386]
              tunnel: w5281 -> [_ w5381]
              tunnel: w5280 -> [_ _]
              tunnel: w5274 -> [w5291 w5374]
              tunnel: w5273 -> [w5290 w5375]
              tunnel: w5272 -> [_ w5373]
              tunnel: w5268 -> [_ w5372]
              tunnel: w5267 -> [_ w5296]
              tunnel: w5266 -> [_ w5365]
              tunnel: w5265 -> [_ w5312]
              tunnel: w5264 -> [w5287 w5329]
              tunnel: w5263 -> [w5288 w5328]
              tunnel: w5262 -> [_ w5325]
              tunnel: w5261 -> [_ w5323]
              frame False {
                w5289 = FALSE
                n3367 = Close File(refnum=w5293) -> ()  [unwired: 1 in, 2 out]
                n3368 = case shown="True" w5290 {
                  tunnel: w5291 -> [_ w5295]
                  frame False {
                  }
                  frame True {
                    n3369 = Close File(refnum=w5295) -> ()  [unwired: 1 in, 2 out]
                  }
                }
                n3370 = case shown="True" w5287 {
                  tunnel: w5288 -> [_ w5294]
                  frame False {
                  }
                  frame True {
                    n3371 = Close File(refnum=w5294) -> ()  [unwired: 1 in, 2 out]
                  }
                }
                n3372 = local write "Raster Scanning..."(w5289) -> ()
                n3373 = local write "Calibrating Trap..."(w5289) -> ()
                n3374 = call <vilib>:"Beep.vi"() -> ()  [unwired: 3 in, 9 out]
                n3375 = local write "Stop Saving"(w5289) -> ()
                "Saving..." <- w5289
              }
              frame True {
                n3376 = local read "Calibrating Trap..."() -> (w5376:bool)
                n3377 = case "Write fl. data" shown="True" w5375 {
                  tunnel: w5374 -> [_ w5410]
                  tunnel: w5373 -> [_ w5409]
                  frame False {
                  }
                  frame True {
                    n3378 = Write to Binary File(file (use dialog)=w5410, data=w5409, 5:FALSE ("prepend array or string size? (T)"), 9:T32."big-endian, network order" ("byte order (0:big-endian, network order)")) -> ()  [unwired: 1 in, 4 out]
                  }
                }
                n3379 = Greater?(x="Save ave N", y=1.0) -> (0:w5379:bool)
                n3380 = Not(x=w5376) -> (.not. x?=w5378:bool)
                n3381 = And(x=w5378, y=w5379) -> (x .and. y?=w5326:bool)
                n3382 = case shown="True" w5326 {
                  tunnel: w5325 -> [w5390 w5401]
                  tunnel: [w5390 w5393] -> w5324
                  tunnel: "Save ave N" -> [_ w5394]
                  frame False {
                  }
                  frame True {
                    w5391 = 2 ("dimension size")
                    n3383 = Array Size(array=w5401) -> (size(s)=w5395:i32)
                    n3384 = Divide(x=w5395, y=w5391) -> (x/y=w5399:dbl)
                    n3385 = Reshape Array(w5401, w5399, w5391) -> (w5400:u64[][])
                    n3386 = Transpose 2D Array(2D array=w5400) -> (transposed array=w5398:u64[][])
                    n3387 = for {
                      tunnel: w5398 -> [w5403] mode=indexing
                      tunnel: [w5402] -> w5392 mode=indexing
                      tunnel: w5394 -> [w5404]
                      workers-P: _ -> [_]
                      n3388 = call "downsample 1D array - U64.vi"("Ave N"=w5404, "Array In"=w5403) -> ("Array Out"=w5402:u64[])  [unwired: 1 in]
                    }
                    n3389 = Transpose 2D Array(2D array=w5392) -> (transposed array=w5397:u64[][])
                    n3390 = Divide(x=w5395, y=w5394) -> (x/y=w5396:dbl)
                    n3391 = Reshape Array(w5397, w5396) -> (w5393:u64[])
                  }
                }
                n3392 = case shown="True" w5326 {
                  tunnel: w5381 -> [w5413 w5425]
                  tunnel: [w5413 w5417] -> w5377
                  tunnel: "Save ave N" -> [_ w5418]
                  tunnel: w5372 -> [_ w5416]
                  frame False {
                  }
                  frame True {
                    n3393 = Array Size(array=w5425) -> (size(s)=w5419:i32)
                    n3394 = Array Size(array=w5416) -> (size(s)=w5415:i32)
                    n3395 = Divide(x=w5419, y=w5415) -> (x/y=w5423:dbl)
                    n3396 = Reshape Array(w5425, w5423, w5415) -> (w5424:i16[][])
                    n3397 = Transpose 2D Array(2D array=w5424) -> (transposed array=w5422:i16[][])
                    n3398 = for {
                      tunnel: w5422 -> [w5428] mode=indexing
                      tunnel: [w5427] -> w5414 mode=indexing
                      tunnel: w5418 -> [w5426]
                      workers-P: _ -> [_]
                      n3399 = call "downsample 1D array - I16.vi"("Ave N"=w5426, "Array In"=w5428) -> ("Array Out"=w5427:i16[])  [unwired: 1 out]
                    }
                    n3400 = Transpose 2D Array(2D array=w5414) -> (transposed array=w5421:i16[][])
                    n3401 = Divide(x=w5419, y=w5418) -> (x/y=w5420:dbl)
                    n3402 = Reshape Array(w5421, w5420) -> (w5417:i16[])
                  }
                }
                n3403 = Index Array(array=w5312, index=2) -> (element=w5313:waveform(dbl))
                n3404 = Index Array(array=w5312, index=1) -> (element=w5346:waveform(dbl))
                n3405 = Index Array(array=w5312, index=0) -> (element=w5348:waveform(dbl))
                n3406 = Unbundle By Name(w5313) -> ("Y"=w5315:dbl[])
                n3407 = Unbundle By Name(w5346) -> ("Y"=w5350:dbl[])
                n3408 = Unbundle By Name(w5348) -> ("Y"=w5358:dbl[])
                n3409 = case "Write trap pos. data" shown="True" w5329 {
                  tunnel: w5328 -> [_ w5406]
                  tunnel: w5324 -> [_ w5405]
                  frame False {
                  }
                  frame True {
                    n3410 = Write to Binary File(file (use dialog)=w5406, data=w5405, 5:FALSE ("prepend array or string size? (T)"), 9:T32."big-endian, network order" ("byte order (0:big-endian, network order)")) -> ()  [unwired: 1 in, 4 out]
                  }
                }
                n3411 = Write to Binary File(file (use dialog)=w5384, data=w5377, 5:FALSE ("prepend array or string size? (T)"), 9:T32."big-endian, network order" ("byte order (0:big-endian, network order)")) -> ()  [unwired: 1 in, 4 out]
                n3412 = feedback #36(w5315) -> (w5316:dbl[])
                n3413 = Build Array (concatenate)(w5316, w5315) -> (w5311:dbl[])
                n3414 = Select(t=w5315, s=w5296, f=w5311) -> (s? t:f=w5301:dbl[])
                n3415 = feedback-in #36(w5301) -> ()
                n3416 = feedback #37(w5350) -> (w5352:dbl[])
                n3417 = Build Array (concatenate)(w5352, w5350) -> (w5351:dbl[])
                n3418 = Select(t=w5350, s=w5296, f=w5351) -> (s? t:f=w5340:dbl[])
                n3419 = feedback-in #37(w5340) -> ()
                n3420 = feedback #38(w5358) -> (w5371:dbl[])
                n3421 = Build Array (concatenate)(w5371, w5358) -> (w5370:dbl[])
                n3422 = Select(t=w5358, s=w5296, f=w5370) -> (s? t:f=w5345:dbl[])
                n3423 = feedback-in #38(w5345) -> ()
                n3424 = Divide(x=w5385, y=w5386) -> (x/y=w5388:dbl)
                n3425 = Multiply(x=w5388, y=100.0) -> (x*y=w5387:dbl)
                n3426 = Build Array(w5345, w5340, w5301) -> (→"Saved APD":dbl[][])
                n3427 = Array Size(array=w5345) -> (size(s)=w5363:i32)
                n3428 = Unbundle By Name(w5365) -> ("Y"=w5369:dbl[])
                n3429 = Subtract(x=w5363, y="N pts to average") -> (x-y=w5298:i32)
                n3430 = Multiply(x="N pts to average", y=u16 2) -> (x*y=w5341:u16)
                n3431 = Subtract(x=w5363, y=w5341) -> (x-y=w5299:i32)
                n3432 = feedback #39(w5369) -> (w5368:dbl[])
                n3433 = Build Array (concatenate)(w5368, w5369) -> (w5367:dbl[])
                n3434 = Select(t=w5369, s=w5296, f=w5367) -> (s? t:f=w5366:dbl[])
                "Trap Delta Graph" <- w5366
                n3435 = feedback-in #39(w5366) -> ()
                n3436 = Array Subset(array=w5345, index=w5298, length="N pts to average") -> (w5362:dbl[])
                n3437 = Array Subset(array=w5345, index=w5299, length="N pts to average") -> (w5361:dbl[])
                n3438 = Array Subset(array=w5340, index=w5298, length="N pts to average") -> (w5343:dbl[])
                n3439 = Array Subset(array=w5340, index=w5299, length="N pts to average") -> (w5342:dbl[])
                n3440 = Array Subset(array=w5301, index=w5298, length="N pts to average") -> (w5310:dbl[])
                n3441 = Array Subset(array=w5301, index=w5299, length="N pts to average") -> (w5309:dbl[])
                n3442 = Index Array(array=w5323, index=0) -> (element=w5321:waveform(dbl))
                n3443 = call-poly <vilib>:"Mean.vi"("X"=w5362) -> ("mean"=w5360:dbl)  [unwired: 1 out]
                n3444 = call-poly <vilib>:"Mean.vi"("X"=w5343) -> ("mean"=w5339:dbl)  [unwired: 1 out]
                n3445 = call-poly <vilib>:"Mean.vi"("X"=w5361) -> ("mean"=w5359:dbl)  [unwired: 1 out]
                n3446 = call-poly <vilib>:"Mean.vi"("X"=w5342) -> ("mean"=w5338:dbl)  [unwired: 1 out]
                n3447 = call-poly <vilib>:"Mean.vi"("X"=w5310) -> ("mean"=w5308:dbl)  [unwired: 1 out]
                n3448 = call-poly <vilib>:"Mean.vi"("X"=w5309) -> ("mean"=w5307:dbl)  [unwired: 1 out]
                n3449 = Unbundle By Name(w5321) -> ("Y"=w5319:dbl[])
                n3450 = Subtract(x=w5339, y=w5338) -> (x-y=w5330:dbl)
                "Delta Fl. 2" <- w5330
                n3451 = Subtract(x=w5308, y=w5307) -> (x-y=w5302:dbl)
                "Delta Fl. 3" <- w5302
                n3452 = Subtract(x=w5360, y=w5359) -> (x-y=w5357:dbl)
                "Delta Fl. 1" <- w5357
                n3453 = feedback #40(w5319) -> (w5318:dbl[])
                n3454 = Build Array (concatenate)(w5318, w5319) -> (w5320:dbl[])
                n3455 = Initialize Array(w5357, 1 ("dimension size")) -> (w5354:dbl[])
                n3456 = Initialize Array(w5330, 1 ("dimension size")) -> (w5335:dbl[])
                n3457 = Initialize Array(w5302, 1 ("dimension size")) -> (w5304:dbl[])
                n3458 = Select(t=w5319, s=w5296, f=w5320) -> (s? t:f=w5317:dbl[])
                "Saved trap pos" <- w5317
                n3459 = feedback-in #40(w5317) -> ()
                n3460 = feedback #41(w5354) -> (w5355:dbl[])
                n3461 = Build Array (concatenate)(w5355, w5354) -> (w5353:dbl[])
                n3462 = feedback #42(w5335) -> (w5336:dbl[])
                n3463 = feedback #43(w5304) -> (w5305:dbl[])
                n3464 = Build Array (concatenate)(w5336, w5335) -> (w5334:dbl[])
                n3465 = Build Array (concatenate)(w5305, w5304) -> (w5303:dbl[])
                n3466 = Select(t=w5354, s=w5296, f=w5353) -> (s? t:f=w5333:dbl[])
                n3467 = feedback-in #41(w5333) -> ()
                n3468 = Select(t=w5335, s=w5296, f=w5334) -> (s? t:f=w5332:dbl[])
                n3469 = feedback-in #42(w5332) -> ()
                n3470 = Select(t=w5304, s=w5296, f=w5303) -> (s? t:f=w5297:dbl[])
                n3471 = feedback-in #43(w5297) -> ()
                n3472 = Build Array(w5333, w5332, w5297) -> (→"Save APD Deriv":dbl[][])
              }
            }
            "Progress" <- w5278
            "Progress 2" <- w5278
          }
        }
      }
    }
    n3473 = local read "wait to reset values"() -> (w3911:bool)
    n3474 = Not(x=w3909) -> (.not. x?=w3912:bool)
    n3475 = And(x=w3912, y=w3911) -> (x .and. y?=w3913:bool)
    n3476 = case "Part of MCL raster scanning: returns to initial positions after scan done" shown="True" w3913 {
      tunnel: w3676 -> [w4801 w4808]
      tunnel: [w4801 w4807] -> w3915
      tunnel: w3675 -> [w4800 w4806]
      tunnel: [w4800 w4805] -> w3910
      frame False {
      }
      frame True {
        w4816 = 10.0 ("y")
        w4815 = 32767.0 ("y")
        # "to return scan values\nafter a synchronous \nAOM scan"
        n3477 = local read "AO2"() -> (w4809:dbl)
        n3478 = local read "AO1"() -> (w4810:dbl)
        n3479 = local write "wait to reset values"(FALSE ("wait to reset values")) -> ()
        n3480 = Multiply(x=w4810, y=w4815) -> (x*y=w4812:dbl)
        n3481 = Multiply(x=w4809, y=w4815) -> (x*y=w4814:dbl)
        n3482 = Divide(x=w4812, y=w4816) -> (x/y=w4811:dbl)
        n3483 = Divide(x=w4814, y=w4816) -> (x/y=w4813:dbl)
        n3484 = To Word Integer(number=w4811) -> (16bit integer=w4817:i16)
        n3485 = To Word Integer(number=w4813) -> (16bit integer=w4818:i16)
        n3486 = local read "Total Counts (ticks)"() -> (w4802:u16)
        n3487 = xnode "Read/Write Control"("FPGA VI Reference In"=w4808, "error in"=w4806, "AO1"=w4817, "AO2"=w4818, "MCL count"=w4802) -> ("FPGA VI Reference Out"=w4807:T24, "error out"=w4805:errorcluster)
        n3488 = local read "Scan Range (V)\n(of steps)"() -> (w4803:dbl)
        n3489 = property on="Scan Range (V)\n(of steps)" class="DigNum (strict)"("Val(Sgnl)"=w4803) -> ()  [unwired: 2 in, 2 out]
      }
    }
    n3490 = case shown="True" "Sound ON" {
      tunnel: [w3929 w3974] -> w3597
      tunnel: w3596 -> [w3929 w3973]
      tunnel: w3594 -> [_ _]
      tunnel: w3572 -> [_ w3932]
      tunnel: w3593 -> [_ _]
      tunnel: w3592 -> [_ w3943]
      tunnel: w3591 -> [_ w3953]
      frame False {
      }
      frame True {
        n3491 = Index Array(array=w3932, index="Data channel to sound") -> (element=w3931:waveform(dbl))
        "Waveform Graph 2" <- w3931
        n3492 = Unbundle By Name(w3931) -> ("dt"=w3957:dbl, "Y"=w3955:dbl[])
        n3493 = Array Size(array=w3955) -> (size(s)=w3956:i32)
        "N data samples" <- w3956
        n3494 = for "Data time base" {
          N: w3956 -> [_]
          tunnel: [w3978] -> w3958 mode=indexing
          i -> [w3978]
        }
        n3495 = Multiply(x=w3957, y=w3958) -> (x*y=w3954:dbl[])
        n3496 = Compound Arithmetic op=MULTIPLY(6.283185307179586, "Carrier Frequency (Hz)", w3953) -> (w3970:dbl[])
        n3497 = call <vilib>:"Interpolate 1D.vi"("X is monotonic"=TRUE, "xi"=w3953, "X"=w3954, "Y"=w3955) -> ("yi"=w3951:dbl[])  [unwired: 5 in, 2 out]
        n3498 = Sine(x=w3970) -> (sin(x)=w3959:dbl[])
        n3499 = Add(x=w3951, y="Offset") -> (x+y=w3949:dbl[])
        n3500 = Multiply(x=w3949, y="mult x") -> (x*y=w3947:dbl[])
        n3501 = Add(x="Offset 2", y=w3947) -> (x+y=w3942:dbl[])
        n3502 = Compound Arithmetic op=MULTIPLY(6.283185307179586, "Carrier Frequency (Hz)", w3943, w3942) -> (w3934:dbl[])
        n3503 = for "Cumulative sum" {
          tunnel: [w3977] -> w3940 mode=indexing
          shift-right: [w3977] -> w3937
          shift-left: 0.0 -> [w3976]
          tunnel: w3934 -> [w3975] mode=indexing
          n3504 = Add(x=w3975, y=w3976) -> (x+y=w3977:dbl)
        }
        n3505 = feedback #44(0.0) -> (w3936:dbl)
        n3506 = Add(x=w3940, y=w3936) -> (x+y=w3939:dbl[])
        n3507 = Add(x=w3937, y=w3936) -> (x+y=w3935:dbl)
        n3508 = feedback-in #44(w3935) -> ()
        n3509 = Sine(x=w3939) -> (sin(x)=w3933:dbl[])
        n3510 = Select(t=w3959, s="tone or data", f=w3933) -> (s? t:f=w3965:dbl[])
        n3511 = Multiply(x=w3965, y="Volume") -> (x*y=w3963:dbl[])
        n3512 = Initialize Array(0.0 ("element"), "N initial buffer elements") -> (w3966:dbl[])
        n3513 = Multiply(x="N initial buffer elements", y=w3943) -> (x*y=→"Initial buffer time (s)":dbl)
        n3514 = Build Array (concatenate)(w3966, w3963) -> (w3968:dbl[])
        n3515 = First Call?() -> (First Call?: T/F=w3969:bool)
        n3516 = Select(t=w3968, s=w3969, f=w3963) -> (s? t:f=w3962:dbl[])
        n3517 = call-poly <vilib>:"Sound Output Write.vi"("data"=w3962, "task ID"=w3973) -> ("task ID out"=w3974:T42)  [unwired: 8 in, 1 out]
      }
    }
    n3518 = node-c288() -> ()  [unwired: 2 out]
  }
  n3519 = call <vilib>:"Sound Output Clear.vi"("task ID"=w12) -> ()  [unwired: 10 in, 1 out]
  n3520 = disable-structure shown="Disabled" {
    disable-tunnel: w69 -> [w5430 _]
    disable-tunnel: w68 -> [w5429 _]
    frame Disabled {
      n3521 = VISA Close(VISA resource name=w5430, error in (no error)=w5429) -> (error out=w5431:errorcluster)
      n3522 = call <vilib>:"Simple Error Handler.vi"("error in (no error)"=w5431) -> ()  [unwired: 1 in, 8 out]
    }
    frame Enabled {
    }
  }
  n3523 = node-c288(w75) -> ()  [unwired: 1 out]
  n3524 = node-c288(w84) -> ()  [unwired: 1 out]
  n3525 = flat-sequence {
    tunnel: w91 -> [w5435]
    tunnel: w92 -> [w5436]
    tunnel: [w5434] -> w90
    tunnel: [w5433] -> w89
    tunnel: w88 -> [_]
    tunnel: w86 -> [_]
    tunnel: w81 -> [_]
    tunnel: w90 -> [w5437]
    tunnel: w89 -> [w5438]
    frame #0 {
      w5432 = FALSE ("AI to FIFO")
      n3526 = xnode "Read/Write Control"("FPGA VI Reference In"=w5436, "error in"=w5435, "AI to FIFO"=w5432, "APD to FIFO"=w5432) -> ("FPGA VI Reference Out"=w5434:T24, "error out"=w5433:errorcluster)
    }
    frame #1 {
      n3527 = xnode "Close FPGA VI Reference"("FPGA VI Reference In"=w5437, "error in"=w5438) -> ("error out"=→"error out":errorcluster)
    }
  }
